vi "UHR-Fleezers Control (host) - Avogadro v3.vi"() -> ()   [LabVIEW 2014] (continued)
              }
            }
          }
          frame "Triggered" {
            n3649 = local read "Trap Trig. (FPGA)"() -> (w5268:bool)
            n3650 = Increment(x=w5271) -> (x+1=w5269:i32)
            n3651 = Greater Or Equal?(x=w5269, y="Fl. ON time (n)") -> (x >= y?=w5267:bool)
            n3652 = Select(t="Wait for trigger", s=w5267, f="Triggered" ("t")) -> (s? t:f=w5272:string)
            n3653 = And(x=w5267, y=w5268) -> (x .and. y?=w5264:bool)
            n3654 = case shown="True" w5264 {
              tunnel: w5266 -> [_ w5276]
              tunnel: w5265 -> [_ w5275]
              frame False {
              }
              frame True {
                n3655 = xnode "Read/Write Control"("FPGA VI Reference In"=w5276, "error in"=w5275, "FPGA Trap Trig"=TRUE) -> ()  [unwired: 2 out]
              }
            }
            n3656 = case shown="True" w5267 {
              frame False {
              }
              frame True {
                w5278 = FALSE ("Value (Signaling)")
                n3657 = local write "Triggered"(w5278) -> ()
                n3658 = local write "Waiting"(TRUE ("Waiting")) -> ()
                n3659 = property on="Vortran Laser ON" class="Bool (strict)"("Val(Sgnl)"=w5278) -> ()  [unwired: 2 in, 2 out]
              }
            }
          }
          frame "Do nothing" {
          }
          frame "Initialize", Default {
            n3660 = Increment(x=w5289) -> (x+1=w5293:i32)
            n3661 = Select(t=1, s=w5282, f=w5293) -> (s? t:f=w5283:i32)
            n3662 = feedback #23(w5291) -> (w5297:dbl[])
            n3663 = Build Array (concatenate)(w5291, w5297) -> (w5290:dbl[])
            n3664 = Greater Or Equal?(x=w5283, y="Wait to get offset (n)") -> (x >= y?=w5286:bool)
            n3665 = Select(t=w5291, s=w5282, f=w5290) -> (s? t:f=w5292:dbl[])
            n3666 = feedback-in #23(w5292) -> ()
            n3667 = call-poly <vilib>:"Mean.vi"("X"=w5292) -> ("mean"=w5287:dbl)  [unwired: 1 out]
            n3668 = local write "Mean T1 Position\nto compare (nm)"(w5287) -> ()
            n3669 = case shown="True" w5282 {
              tunnel: w5285 -> [_ w5303]
              tunnel: w5284 -> [_ w5302]
              frame False {
              }
              frame True {
                w5299 = FALSE ("FPGA Trap Trig")
                n3670 = xnode "Read/Write Control"("FPGA VI Reference In"=w5303, "error in"=w5302, "FPGA Trap Trig"=w5299) -> ("FPGA VI Reference Out"=w5301:T41, "error out"=w5300:errorcluster)
                n3671 = xnode "Read/Write Control"("FPGA VI Reference In"=w5301, "error in"=w5300, "TTrig?"=w5299) -> ()  [unwired: 2 out]
              }
            }
            n3672 = Select(t="Wait for trigger", s=w5286, f="Initialize") -> (s? t:f=w5294:string)
            n3673 = case shown="True" w5286 {
              tunnel: w5287 -> [_ w5306]
              tunnel: w5285 -> [_ w5315]
              tunnel: w5284 -> [_ w5314]
              frame False {
                n3674 = local write "Waiting"(FALSE ("Waiting")) -> ()
                "Initializing" <- TRUE ("Initializing")
              }
              frame True {
                n3675 = local read "Threshold (nm)"() -> (w5318:dbl)
                n3676 = local read "AOM X Cal (nm/MHz)"() -> (w5317:dbl)
                n3677 = Add(x=w5306, y=w5318) -> (x+y=w5319:dbl)
                n3678 = Divide(x=w5319, y=w5317) -> (x/y=w5316:dbl)
                n3679 = call "IR AOM freq to word.vi"("Frequency In (MHz)"=w5316) -> ("Frequency Word Out (double)"=w5313:dbl)
                n3680 = local write "Initializing"(FALSE ("Initializing")) -> ()
                n3681 = local write "Waiting"(TRUE ("Waiting")) -> ()
                n3682 = To Quad Integer(1:w5313) -> (0:w5312:i64)
                n3683 = xnode "Read/Write Control"("FPGA VI Reference In"=w5315, "error in"=w5314, "FPGA TTrig Thresh"=w5312) -> ("FPGA VI Reference Out"=w5309:T41, "error out"=w5308:errorcluster)
                n3684 = xnode "Read/Write Control"("FPGA VI Reference In"=w5309, "error in"=w5308, "FPGA Trap Trig"=TRUE) -> ()  [unwired: 2 out]
              }
            }
          }
        }
      }
    }
    n3685 = feedback-in #21(w4841) -> ()
    n3686 = feedback-in #22(w4838) -> ()
    n3687 = xnode ("Read/Write Control")("FPGA VI Reference In"=w4633, "error in"=w4900) -> ("FPGA VI Reference Out"=w4630:T41, "error out"=w4826:errorcluster, "AI2 Y Sum Set 1"=w4942:i16, "AI2 Y Sum Set 2"=w4941:i16, "AI1 X Set 1"=w4857:fxp<+/-,16,1>, "AI1 X Set 2"=w4856:fxp<+/-,16,1>, "Trap Pos FB Int Signal"=→"Trap Pos FB Int Signal":fxp<+/-,24,9>, "Trap Pos FB Int-Norm Signal"=→"Trap Pos FB Int-Norm Signal":fxp<+/-,16,1>, "Trap Pos FB Action"=w4850:i64, "Scanning"=→"AOD Scanning":bool, "Scan I"=→"AOD Scan I":u64, "Scanning MCL"=w4944:bool, "Scan I (MCL)"=→"MCL Scan I":u64, "Green FB Sum"=w4907:i16, "Trap Pos FB Action"=w4824:i64, "TTrig Fin Thresh"=w4820:i64, "Red FB Intensity"=w4812:i16, "Blue Intensity"=w4807:i16, "BD1 Frequency Out 1"=w4772:u64)
    "MCL Scanning" <- w4944
    "Trap Pos FB Action" <- w4850
    n3688 = Divide(x=w4812, y=3276.7) -> (x/y=w4811:dbl)
    "Red laser intensity (V)" <- w4811
    n3689 = Divide(x=w4807, y=3276.7) -> (x/y=w4806:dbl)
    "Blue laser intensity (V)" <- w4806
    n3690 = Divide(x=w4907, y=3276.7) -> (x/y=w4810:dbl)
    "Green laser intensity (V)" <- w4810
    n3691 = local read "FB Trig Integrate"() -> (w4818:u32)
    n3692 = Divide(x=w4824, y=w4818) -> (x/y=w4817:dbl)
    "TTrig Sig (Int)" <- w4817
    n3693 = Bundle(w4810, w4811, w4806) -> (→"Fluorescence laser intensities plot":cluster{dbl, dbl, dbl})  [unwired: 1 in]
    n3694 = Divide(x=w4820, y=w4818) -> (x/y=w4815:dbl)
    "TTrig Fin Thresh (Int)" <- w4815
    n3695 = local read "AOM X Cal (nm/MHz)"() -> (w4823:dbl)
    n3696 = local read "AI2 (V)"() -> (w4943:cluster{"Set 1":dbl, "Set 2":dbl})
    n3697 = Bundle By Name(cluster=w4943, "Set 1"=w4942, "Set 2"=w4941) -> (w4774:cluster{"Set 1":dbl, "Set 2":dbl})
    n3698 = Divide(x=w4850, y=327.67) -> (x/y=→"Action (%)":dbl)
    n3699 = case shown="True" "Semi Passive Mode" {
      tunnel: w4680 -> [_ w5091]
      frame False {
      }
      frame True {
        n3700 = local read "Target Force (pN)"() -> (w5089:dbl)
        n3701 = Less?(x="Jump Force (pN)", y=w5089) -> (x < y?=w5087:bool)
        n3702 = case shown="False" w5087 {
          tunnel: "Jump Force (pN)" -> [w5097 w5100]
          tunnel: w5091 -> [w5096 w5099]
          tunnel: [w5095 w5098] -> w5090
          frame False {
            n3703 = Less?(x=w5097, y=w5096) -> (x < y?=w5095:bool)
          }
          frame True {
            n3704 = Greater?(x=w5100, y=w5099) -> (0:w5098:bool)
          }
        }
        n3705 = case shown="False" w5090 {
          frame False {
            n3706 = local read "Trap Pos. FB ON"() -> (w5092:bool)
            n3707 = case shown="False" w5092 {
              frame False {
              }
              frame True {
                n3708 = property on="Trap Pos. FB ON" class="Bool (strict)"("Val(Sgnl)"=FALSE) -> ()  [unwired: 2 in, 2 out]
              }
            }
          }
          frame True {
            n3709 = property on="Trap Pos. FB ON" class="Bool (strict)"("Val(Sgnl)"=TRUE) -> ()  [unwired: 2 in, 2 out]
          }
        }
      }
    }
    n3710 = local read "Trap X (AI1)"() -> (w4870:T19)
    n3711 = call "IR AOM word double to freq.vi"("Frequency Word In (double)"=w4815) -> ("Frequency Out (MHz)"=w4814:dbl)
    n3712 = call "IR AOM word double to freq.vi"("Frequency Word In (double)"=w4817) -> ("Frequency Out (MHz)"=w4816:dbl)
    n3713 = Divide(x=w4774, y=3276.7) -> (x/y=w4939:cluster{"Set 1":dbl, "Set 2":dbl})
    n3714 = Multiply(x=w4816, y=w4823) -> (x*y=w4822:dbl)
    "TTrig Sig (nm)" <- w4822
    n3715 = Multiply(x=w4814, y=w4823) -> (x*y=w4821:dbl)
    "TTrig Fin Thresh (nm)" <- w4821
    n3716 = local write "AI2 (V)"(w4939) -> ()
    n3717 = Bundle(cluster=w4870, "Trap 1"=w4857, "Trap 2"=w4856) -> (→"Trap X (AI1)":T19)
    n3718 = local read "Trap Pos. FB ON"() -> (w4765:bool)
    n3719 = local read "Dynamic Force FB (ronen)"() -> (w4766:bool)
    n3720 = Bundle(w4822, w4821) -> (→"TTrig":cluster{dbl, dbl})  [unwired: 1 in]
    n3721 = Compound Arithmetic op=AND(w4766, "Real time Offset file correction for setpoint", w4765) -> (w4767:bool)
    n3722 = case shown="True" w4767 {
      tunnel: w4772 -> [_ _]
      tunnel: w4703 -> [_ w5119]
      tunnel: w4630 -> [_ w5102]
      frame False {
      }
      frame True {
        # "Changed by Ronen - real time update of set point\naccording to offset file"
        n3723 = local read "T1 calibration"() -> (w5114:T12)
        n3724 = local read "Offset file step size"() -> (w5121:dbl)
        n3725 = local read "Setpoint offset\ncorrection values"() -> (w5118:dbl[])
        n3726 = Multiply(x="Target Force (pN)", y=2.0) -> (x*y=w5115:dbl)
        n3727 = local read "Negate Diff?"() -> (w5103:bool)
        n3728 = Unbundle By Name(w5114) -> ("alpha_x (nm/V)"=w5113:dbl, "kappa_x (pN/nm)"=w5112:dbl)
        n3729 = Divide(x=w5119, y=w5121) -> (x/y=w5122:dbl)
        n3730 = To Long Integer(number=w5122) -> (32bit integer=w5120:i32)
        n3731 = Index Array(array=w5118, index=w5120) -> (element=w5105:dbl)
        n3732 = Multiply(x=w5113, y=w5112) -> (x*y=w5111:dbl)
        n3733 = Select(t=1, s=w5103, f=-1) -> (s? t:f=w5106:i32)
        n3734 = Divide(x=w5115, y=w5111) -> (x/y=w5110:dbl)
        n3735 = Multiply(x=w5106, y=w5105) -> (x*y=w5104:dbl)
        n3736 = Add(x=w5110, y=w5104) -> (x+y=w5109:dbl)
        n3737 = To Fixed-Point(number=w5109) -> (fixed-point=w5101:fxp<+/-,16,1>)  [unwired: 1 in]
        "Actual Setpoint" <- w5101
        n3738 = xnode "Read/Write Control"("FPGA VI Reference In"=w5102, "Trap Pos. FB SP"=w5101) -> ()  [unwired: 1 in, 2 out]
      }
    }
    n3739 = local read "All FB On/Off"() -> (w4773:bool)
    n3740 = case shown="True" w4773 {
      tunnel: w4630 -> [_ w5146]
      frame False {
      }
      frame True {
        n3741 = local read "X RF Amplitude Limits (%)"() -> (w5145:T27)
        n3742 = xnode "Read/Write Control"("FPGA VI Reference In"=w5146) -> ("BD1 amplitude 1 out"=w5137:u16, "BD1 amplitude 2 out"=w5129:u16)  [unwired: 1 in, 2 out]
        n3743 = Unbundle By Name(w5145) -> ("Maximum"=w5128:dbl)
        n3744 = Scale By Power Of 2(n=i16 12, x=ext 1.0) -> (x*2^n=w5141:ext)
        n3745 = Scale By Power Of 2(n=i16 12, x=ext 1.0) -> (x*2^n=w5133:ext)
        n3746 = Subtract(x=w5141, y=ext 1.0) -> (x-y=w5143:ext)
        n3747 = Subtract(x=w5133, y=ext 1.0) -> (x-y=w5131:ext)
        n3748 = Multiply(x=w5137, y=ext 100.0) -> (x*y=w5144:ext)
        n3749 = Multiply(x=w5129, y=ext 100.0) -> (x*y=w5130:ext)
        n3750 = Divide(x=w5144, y=w5143) -> (x/y=w5124:ext)
        "T1 feedback amplitude" <- w5124
        n3751 = Divide(x=w5130, y=w5131) -> (x/y=w5123:ext)
        "T2 feedback amplitude" <- w5123
        n3752 = Greater?(x=w5123, y=w5128) -> (0:w5126:bool)
        n3753 = Greater?(x=w5124, y=w5128) -> (0:w5127:bool)
        n3754 = Or(x=w5127, y=w5126) -> (x .or. y?=w5125:bool)
        n3755 = case shown="True" w5125 {
          frame False {
          }
          frame True {
            n3756 = property on="All FB On/Off" class="Bool (strict)"("Val(Sgnl)"=FALSE) -> ()  [unwired: 2 in, 2 out]
          }
        }
      }
    }
    n3757 = flat-sequence "To save data" {
      tunnel: [w5865] -> w4962
      tunnel: [w5866] -> w4961
      tunnel: w4924 -> [w5859]
      tunnel: w4646 -> [w5863]
      tunnel: ["Save Calibration"] -> w4936
      tunnel: w4755 -> [w5862]
      tunnel: [w5855] -> w4933
      tunnel: [w5852] -> w4932
      tunnel: [w5849] -> w4931
      tunnel: w4923 -> [w5851]
      tunnel: w4711 -> [w5845]
      tunnel: [w5845] -> w4894
      tunnel: ["Start Saving"] -> w4879
      tunnel: [w5840] -> w4846
      tunnel: [w5839] -> w4845
      tunnel: [w5836] -> w4778
      tunnel: [w5832] -> w4771
      tunnel: w4962 -> [w6199]
      tunnel: w4961 -> [w6198]
      tunnel: w4756 -> [w6197]
      tunnel: w4936 -> [w6196]
      tunnel: w4933 -> [w6194]
      tunnel: w4932 -> [w6193]
      tunnel: w4931 -> [w6192]
      tunnel: w4750 -> [w6191]
      tunnel: w4754 -> [w6190]
      tunnel: w4894 -> [w6189]
      tunnel: w4879 -> [w6188]
      tunnel: w4634 -> [w6187]
      tunnel: w4805 -> [w6186]
      tunnel: w4846 -> [w6185]
      tunnel: w4845 -> [w6184]
      tunnel: w4707 -> [w6183]
      tunnel: w4716 -> [w6182]
      tunnel: w4753 -> [w6181]
      tunnel: w4778 -> [w6180]
      tunnel: w4771 -> [w6179]
      frame #0 {
        # "Changed by Ronen - we don't have a database so we disabled this"
        n3758 = Or(x="Save N Sets", y="Start Saving") -> (x .or. y?=w5846:bool)
        n3759 = To Double Precision Float(number=w5862) -> (double precision float=w5856:dbl)
        n3760 = Build Array(w5846, "Save Calibration", w5859, w5851, "Flow Cal") -> (w5861:bool[])
        n3761 = Compound Arithmetic op=OR("Save Calibration", w5859, w5846, w5851, "Flow Cal") -> (w5864:bool)
        n3762 = Boolean Array To Number(Boolean array=w5861) -> (number=w5858:u32)
        n3763 = feedback #24(FALSE ("Save APD Data\nwith Trap Data")) -> (w5841:bool)
        n3764 = feedback #25(refnum<k0> refnum) -> (w5867:refnum<file>)
        n3765 = feedback #26(FALSE ("Save APD Data\nwith Trap Data")) -> (w5850:bool)
        n3766 = feedback #27(0) -> (w5869:i32)
        n3767 = feedback #28() -> (w5857:u32)  [unwired: 1 out]
        n3768 = feedback #29(refnum<k0> refnum) -> (w5837:refnum<file>)
        n3769 = feedback #30(refnum<k0> refnum) -> (w5843:refnum<file>)
        n3770 = feedback #31(refnum<k0> refnum) -> (w5833:refnum<file>)
        n3771 = feedback #32(refnum<k0> refnum) -> (w5853:refnum<file>)
        n3772 = case shown="True" w5864 {
          tunnel: [w5878 1] -> w5865
          tunnel: w5869 -> [w5880 _]
          tunnel: [w5879 w5912] -> w5866
          tunnel: w5867 -> [w5879 _]
          tunnel: w5863 -> [_ w5930]
          tunnel: w5856 -> [_ w5928]
          tunnel: w5858 -> [_ w5931]
          tunnel: [w5877 w5911] -> w5855
          tunnel: w5857 -> [w5877 _]
          tunnel: [w5876 w5909] -> w5852
          tunnel: w5853 -> [w5876 _]
          tunnel: [w5875 w5908] -> w5849
          tunnel: w5850 -> [w5875 _]
          tunnel: "Start Saving" -> [_ w5906]
          tunnel: w5845 -> [_ w5905]
          tunnel: [w5874 w5898] -> w5839
          tunnel: w5843 -> [w5874 _]
          tunnel: [w5873 w5897] -> w5840
          tunnel: w5841 -> [w5873 _]
          tunnel: [w5872 w5883] -> w5836
          tunnel: w5837 -> [w5872 _]
          tunnel: [w5871 w5881] -> w5832
          tunnel: w5833 -> [w5871 _]
          frame False {
            n3773 = Increment(x=w5880) -> (x+1=w5878:i32)
          }
          frame True {
            w5882 = FALSE ("Start Saving")
            w5907 = 10.0  # File Version
            w5914 = FALSE ("prepend array or string size? (T)")
            w5913 = T54."big-endian, network order" ("byte order (0:big-endian, network order)")
            # "RG added position values of traps in the saved\nfile for AOD rasters and time series."
            # "Ronen Changed the create file - changed data folder to c:\\Data"
            # "Save trap position\ndata"
            n3774 = Array Size(array=w5905) -> (size(s)=w5904:i32)
            n3775 = To Double Precision Float(number=w5904) -> (double precision float=w5903:dbl)
            n3776 = local read "BD 1 Frequency 1 (MHz)"() -> (w5927:dbl)
            n3777 = local read "BD 2 Frequency 1 (MHz)"() -> (w5926:dbl)
            n3778 = local read "BD 1 Frequency 2 (MHz)"() -> (w5925:dbl)
            n3779 = local read "BD 2 Frequency 2 (MHz)"() -> (w5924:dbl)
            n3780 = local read "BD 1 Frequency 3 (MHz)"() -> (w5923:dbl)
            n3781 = local read "BD 2 Frequency 3 (MHz)"() -> (w5922:dbl)
            n3782 = local write "Flow Cal"(w5882) -> ()
            n3783 = local write "Save Calibration"(w5882) -> ()
            n3784 = local write "Start Saving"(w5882) -> ()
            n3785 = Build Array("Save APD Data\nwith Trap Data", "Save Trap Pos. Data") -> (w5900:bool[])
            n3786 = Boolean Array To Number(Boolean array=w5900) -> (number=w5899:u32)
            n3787 = Build Array(w5927, w5926, w5925, w5924, w5923, w5922) -> (w5921:dbl[])
            n3788 = case shown="1, Default" w5931 {
              tunnel: w5930 -> [w6037 w6064 w6096 w6134 w6171]
              tunnel: w5903 -> [w6042 w6071 w6116 w6153 w6176]
              tunnel: w5928 -> [w6041 w6070 w6115 w6152 w6175]
              tunnel: [w6038 w6066 w6107 w6144 w6172] -> w5919
              tunnel: [w6029 "Cal sets to save" w6097 w6135 w6158] -> w5911
              tunnel: w5921 -> [w6039 w6067 w6109 w6146 w6173]
              tunnel: "Save APD Data\nwith Trap Data" -> [w6036 w6053 w6094 w6132 w6170]
              tunnel: [w6036 w6051 w6094 w6132 w6170] -> w5908
              tunnel: w5907 -> [w6032 w6060 w6092 w6130 w6166]
              tunnel: w5906 -> [w6031 _ _ _ _]
              tunnel: [w6022 w6059 w6091 w6120 w6165] -> w5897
              tunnel: "Save Trap Pos. Data" -> [w6022 w6058 w6091 w6120 w6165]
              tunnel: w5899 -> [w6021 w6057 w6090 w6119 w6164]
              frame 1, Default {
                # "timeseries"
                n3789 = case shown="True" "Profile" {
                  tunnel: [w6045 w6049] -> w6026
                  tunnel: [w6045 w6048] -> w6025
                  tunnel: [w6045 w6047] -> w6024
                  tunnel: [w6045 w6046] -> w6023
                  frame False {
                    w6045 = 0.0 ("f")
                  }
                  frame True {
                    n3790 = local read "Current Position"() -> (w6050:cluster{dbl, dbl, dbl})
                    n3791 = local read "Y change (mm)"() -> (w6046:dbl)
                    n3792 = Unbundle(w6050) -> (w6049:dbl, w6048:dbl, w6047:dbl)
                  }
                }
                n3793 = local read "Save ave N"() -> (w6044:dbl)
                n3794 = local read "AOM X Cal (nm/MHz)"() -> (w6020:dbl)
                n3795 = local read "Piezo Trap X cal (nm/V)"() -> (w6019:dbl)
                n3796 = local read "Piezo Trap Y cal (nm/V)"() -> (w6018:dbl)
                n3797 = local read "Piezo trap x\noffset (V)"() -> (w6017:dbl)
                n3798 = local read "Piezo trap y\noffset (V)"() -> (w6016:dbl)
                n3799 = To Double Precision Float(number=w6021) -> (double precision float=w6035:dbl)
                n3800 = Multiply(x=w6044, y=w6037) -> (x*y=w6043:dbl)
                n3801 = Build Array(w6032, w6037, w6043, w6042, w6041, 0.0 ("f")) -> (w6040:dbl[])
                n3802 = Build Array(w6035, w6026, w6025, w6024, w6023) -> (w6033:dbl[])
                n3803 = Build Array(w6020, w6019, w6018, w6017, w6016) -> (w6015:dbl[])
                n3804 = Select(t=u32 4000000000, s=w6031, f="N sets to save") -> (s? t:f=w6029:u32)
                n3805 = Build Array (concatenate)(w6040, w6039, w6033, w6015) -> (w6038:dbl[])
              }
              frame 2 {
                w6062 = 0.0 ("f")
                w6052 = FALSE ("Save APD Data\nwith Trap Data")
                # "For diagnostics save trap position\ndata during cal"
                # "calibration"
                n3806 = Boolean To (0,1)(Boolean=w6052) -> (0, 1=w6056:i16)
                n3807 = Select(t=w6053, s="Save trap pos with cal", f=w6052) -> (s? t:f=w6051:bool)
                n3808 = Select(t=w6058, s="Save trap pos with cal", f=w6052) -> (s? t:f=w6059:bool)
                n3809 = Select(t=w6057, s="Save trap pos with cal", f=w6056) -> (s? t:f=w6055:u32)
                n3810 = To Double Precision Float(number=w6055) -> (double precision float=w6063:dbl)
                n3811 = Build Array(w6060, w6064, w6064, w6071, w6070, 1.0 ("t")) -> (w6068:dbl[])
                n3812 = Build Array(w6063, w6062, w6062, w6062, w6062) -> (w6061:dbl[])
                n3813 = Build Array (concatenate)(w6068, w6067, w6061) -> (w6066:dbl[])
                "Calibrating Trap..." <- TRUE ("Calibrating...")
              }
              frame 4 {
                # "scan dir (x/y = 0/1)"
                # "cycles/step"
                # "n scans (f/b)"
                # "steps"
                # "freq. range"
                # "AOD raster scan"
                n3814 = local read "MCL offset scanning range (V)"() -> (w6087:T4)
                n3815 = local read "Multiple-MCL offset?"() -> (w6082:bool)
                n3816 = local read "Piezo Trap Y cal (nm/V)"() -> (w6073:dbl)
                n3817 = local read "AOM X Cal (nm/MHz)"() -> (w6075:dbl)
                n3818 = local read "Piezo Trap X cal (nm/V)"() -> (w6076:dbl)
                n3819 = local read "Piezo trap x\noffset (V)"() -> (w6077:dbl)
                n3820 = local read "Piezo trap y\noffset (V)"() -> (w6078:dbl)
                n3821 = local read "Number of F/B Scans (AOD)"() -> (w6101:u16)
                n3822 = Boolean To (0,1)(Boolean="Offset raster?") -> (0, 1=w6080:i16)
                n3823 = call "Make Trap3 position array.vi"("MCL offset scanning range (V)"=w6087) -> ("X Data points"=w6086:u64, "Y data points"=w6085:u64)  [unwired: 3 out]
                n3824 = Boolean To (0,1)(Boolean=w6082) -> (0, 1=w6089:i16)
                n3825 = local read "Cycles/step (AOD)"() -> (w6103:u64)
                n3826 = local read "Scan Range (MHz)"() -> (w6106:dbl)
                n3827 = local read "Scan steps (AOD)"() -> (w6105:u64)
                n3828 = local read "Scan BD"() -> (w6113:bool)
                n3829 = To Double Precision Float(number=w6089) -> (double precision float=w6088:dbl)
                n3830 = local read "Save ave N"() -> (w6118:dbl)
                n3831 = To Double Precision Float(number=w6085) -> (double precision float=w6083:dbl)
                n3832 = Build Array(w6075, w6076, w6073, w6077, w6078) -> (w6074:dbl[])
                n3833 = To Double Precision Float(number=w6086) -> (double precision float=w6084:dbl)
                n3834 = Boolean To (0,1)(Boolean=w6113) -> (0, 1=w6112:i16)
                n3835 = To Double Precision Float(number=w6080) -> (double precision float=w6079:dbl)
                n3836 = To Double Precision Float(number=w6101) -> (double precision float=w6100:dbl)
                n3837 = To Double Precision Float(number=w6105) -> (double precision float=w6104:dbl)
                n3838 = To Double Precision Float(number=w6103) -> (double precision float=w6102:dbl)
                n3839 = To Double Precision Float(number=w6112) -> (double precision float=w6111:dbl)
                n3840 = Multiply(x=w6118, y=w6096) -> (x*y=w6117:dbl)
                n3841 = To Double Precision Float(number=w6090) -> (double precision float=w6095:dbl)
                n3842 = local read "N sets should be saved"() -> (w6098:dbl)
                n3843 = Build Array(w6095, w6088, w6084, w6083, w6079) -> (w6093:dbl[])
                n3844 = Build Array(w6111, w6106, w6104, w6102, w6100) -> (w6108:dbl[])
                n3845 = Build Array(w6092, w6096, w6117, w6116, w6115, 2.0 ("t")) -> (w6110:dbl[])
                n3846 = Build Array (concatenate)(w6110, w6109, w6093, w6108, w6074) -> (w6107:dbl[])
                n3847 = Round Toward +Infinity(x=w6098) -> (ceil(x): smallest int >= x=w6099:dbl)
                n3848 = To Unsigned Long Integer(number=w6099) -> (unsigned 32bit integer=w6097:u32)
              }
              frame 8 {
                w6127 = 0.0 ("f")
                # "MCL raster scan"
                n3849 = local read "Number of scans (MCL)"() -> (w6122:u64)
                n3850 = local read "2D or 1D Scan"() -> (w6124:bool)
                n3851 = local read "Scan lines (y)"() -> (w6121:u64)
                n3852 = local read "Scan Range (V)\n(of steps)"() -> (w6143:dbl)
                n3853 = local read "Fast Scan Dir"() -> (w6150:bool)
                n3854 = local read "Cycles/step (MCL)"() -> (w6140:u64)
                n3855 = local read "Scan steps (MCL)"() -> (w6142:u64)
                n3856 = Select(t=w6121, s=w6124, f=w6122) -> (s? t:f=w6123:u64)
                n3857 = Boolean To (0,1)(Boolean=w6124) -> (0, 1=w6126:i16)
                n3858 = local read "Save ave N"() -> (w6155:dbl)
                n3859 = local read "Initial X"() -> (w6129:dbl)
                n3860 = local read "Initial Y"() -> (w6128:dbl)
                n3861 = To Double Precision Float(number=w6126) -> (double precision float=w6125:dbl)
                n3862 = Boolean To (0,1)(Boolean=w6150) -> (0, 1=w6149:i16)
                n3863 = To Double Precision Float(number=w6123) -> (double precision float=w6138:dbl)
                n3864 = To Double Precision Float(number=w6142) -> (double precision float=w6141:dbl)
                n3865 = To Double Precision Float(number=w6140) -> (double precision float=w6139:dbl)
                n3866 = To Double Precision Float(number=w6149) -> (double precision float=w6148:dbl)
                n3867 = Multiply(x=w6155, y=w6134) -> (x*y=w6154:dbl)
                n3868 = To Double Precision Float(number=w6119) -> (double precision float=w6133:dbl)
                n3869 = local read "N sets should be saved (MCL)"() -> (w6136:dbl)
                n3870 = Build Array(w6133, w6125, w6127, w6127, w6127) -> (w6131:dbl[])
                n3871 = Build Array(w6148, w6143, w6141, w6139, w6138, w6129, w6128) -> (w6145:dbl[])
                n3872 = Build Array(w6130, w6134, w6154, w6153, w6152, 3.0 ("t")) -> (w6147:dbl[])
                n3873 = Round Toward +Infinity(x=w6136) -> (ceil(x): smallest int >= x=w6137:dbl)
                n3874 = Build Array (concatenate)(w6147, w6146, w6131, w6145) -> (w6144:dbl[])
                n3875 = To Unsigned Long Integer(number=w6137) -> (unsigned 32bit integer=w6135:u32)
              }
              frame 16 {
                w6157 = 0.0
                # "Flow calibration - added by Ronen: Number\nof saved sets is distance (1 mm) divided by \nspeed +1.5 spare second divided by the time of\nset measurement, 0.2 sec for 2 set interlace"
                # "timeseries"
                n3876 = local read "Save ave N"() -> (w6178:dbl)
                n3877 = Reciprocal(x=0.0) -> (1/x=w6163:dbl)
                n3878 = Add(x=w6163, y=1.5) -> (x+y=w6161:dbl)
                n3879 = Multiply(x=w6178, y=w6171) -> (x*y=w6177:dbl)
                n3880 = Divide(x=w6161, y=0.2) -> (x/y=w6159:dbl)
                n3881 = To Double Precision Float(number=w6164) -> (double precision float=w6169:dbl)
                n3882 = To Unsigned Long Integer(number=w6159) -> (unsigned 32bit integer=w6158:u32)
                n3883 = Build Array(w6166, w6171, w6177, w6176, w6175, 4.0 ("f")) -> (w6174:dbl[])
                n3884 = Build Array(w6169, w6157, w6157, w6157, w6157) -> (w6167:dbl[])
                n3885 = Build Array (concatenate)(w6174, w6173, w6167) -> (w6172:dbl[])
              }
            }
            n3886 = local read "Index"() -> (w5936:dbl)
            n3887 = call "Create new save file.vi"("Insert"="", "Ext"=".dat", "Index In"=w5936) -> ("Path Out"=w5885:path, "Index Out"=w5910:dbl)
            n3888 = local write "Save file name"(w5885) -> ()
            n3889 = local write "Index"(w5910) -> ()
            n3890 = local write "Save index"(w5910) -> ()
            n3891 = case shown="True" "Save Event Log?" {
              tunnel: w5885 -> [_ w5950]
              tunnel: [refnum<k0> refnum w5949] -> w5883
              frame False {
              }
              frame True {
                (unwired) FALSE ("prepend array or string size? (T)")
                n3892 = Path To String(path=w5950) -> (string=w5961:string)
                n3893 = String Length(string=w5961) -> (length=w5960:i32)
                n3894 = Subtract(x=w5960, y=4) -> (x-y=w5958:i32)
                n3895 = String Subset(string=w5961, length (rest)=w5958) -> (substring=w5957:string)  [unwired: 1 out]
                n3896 = Concatenate Strings(w5957, "_log.txt" ("string")) -> (w5955:string)
                n3897 = String To Path(string=w5955) -> (path=w5951:path)
                n3898 = Open/Create/Replace File(file path (use dialog)=w5951, operation (0:open)=T53."create", access (0:read/write)=enum16{"read/write", "read-only", "write-only"}."write-only") -> (refnum out=w5952:refnum<file>)  [unwired: 1 in, 4 out]
                n3899 = Deny Access(7:w5952) -> (3:w5949:refnum<file>)  [unwired: 1 in, 2 out]
                n3900 = call "write to event log.vi"("log file ref"=w5949, "time"=0.0, "input string"="start log") -> ()  [unwired: 8 in]
              }
            }
            "log file ref" <- w5883
            n3901 = Array Size(array=w5919) -> (size(s)=w5920:i32)
            n3902 = Open/Create/Replace File(file path (use dialog)=w5885, operation (0:open)=T53."create", access (0:read/write)=enum16{"read/write", "read-only", "write-only"}."write-only") -> (refnum out=w5933:refnum<file>)  [unwired: 1 in, 4 out]
            n3903 = local write "Saving..."(TRUE ("Saving...")) -> ()
            n3904 = To Double Precision Float(number=w5920) -> (double precision float=w5918:dbl)
            n3905 = String Length(string="Comment (data description)") -> (length=w5917:i32)
            n3906 = To Double Precision Float(number=w5917) -> (double precision float=w5916:dbl)
            n3907 = Deny Access(7:w5933) -> (3:w5932:refnum<file>)  [unwired: 1 in, 2 out]
            n3908 = Build Array (concatenate)(w5918, w5919, w5916) -> (w5895:dbl[])
            n3909 = case "If fluorescence data to be saved" shown="True" w5908 {
              tunnel: w5885 -> [_ w6014]
              tunnel: [w5984 w5997] -> w5909
              tunnel: [w5984 w5985] -> w5881
              frame False {
                w5984 = refnum<k0> refnum
              }
              frame True {
                w5996 = 0.0
                w5989 = T53."create" ("operation (0:open)")
                w5990 = enum16{"read/write", "read-only", "write-only"}."write-only" ("access (0:read/write)")
                n3910 = local read "APD Integration Time (s)"() -> (w6002:dbl)
                n3911 = local read "N APD Samp/step"() -> (w5995:dbl)
                n3912 = local read "Number of APDs"() -> (w5994:u8)
                n3913 = Path To String(path=w6014) -> (string=w6013:string)
                n3914 = String Length(string=w6013) -> (length=w6012:i32)
                n3915 = Subtract(x=w6012, y=4) -> (x-y=w6010:i32)
                n3916 = String Subset(string=w6013, length (rest)=w6010) -> (substring=w5993:string)  [unwired: 1 out]
                n3917 = Build Array(w6002, w5995, w5994, w5996, w5996, w5996, w5996, w5996) -> (w5999:dbl[])
                n3918 = Concatenate Strings(w5993, "_green.dat") -> (w5991:string)
                n3919 = Concatenate Strings(w5993, "_fl.dat" ("string")) -> (w6008:string)
                n3920 = Array Size(array=w5999) -> (size(s)=w6001:i32)
                n3921 = String To Path(string=w6008) -> (path=w6006:path)
                n3922 = Open/Create/Replace File(file path (use dialog)=w6006, operation (0:open)=w5989, access (0:read/write)=w5990) -> (refnum out=w6007:refnum<file>)  [unwired: 1 in, 4 out]
                n3923 = Deny Access(7:w6007) -> (3:w6003:refnum<file>)  [unwired: 1 in, 2 out]
                n3924 = String To Path(string=w5991) -> (path=w5988:path)
                n3925 = To Double Precision Float(number=w6001) -> (double precision float=w6000:dbl)
                n3926 = Build Array (concatenate)(w6000, w5999) -> (w5998:dbl[])
                n3927 = Write to Binary File(file (use dialog)=w6003, data=w5998, 5:FALSE ("prepend array or string size? (T)"), 9:T54."big-endian, network order" ("byte order (0:big-endian, network order)")) -> (refnum out=w5997:refnum<file>)  [unwired: 1 in, 3 out]
                n3928 = Open/Create/Replace File(file path (use dialog)=w5988, operation (0:open)=w5989, access (0:read/write)=w5990) -> (refnum out=w5986:refnum<file>, error out=w5987:errorcluster)  [unwired: 3 in, 1 out]
                n3929 = Deny Access(4:w5987, 7:w5986) -> (3:w5985:refnum<file>)  [unwired: 1 in, 1 out]
              }
            }
            n3930 = case shown="True" w5897 {
              tunnel: w5885 -> [_ w5969]
              tunnel: [refnum<k0> refnum w5968] -> w5898
              frame False {
              }
              frame True {
                w5964 = 0.0 ("element")
                n3931 = Path To String(path=w5969) -> (string=w5983:string)
                n3932 = Build Array(w5964, w5964, w5964, w5964, w5964, w5964, w5964, w5964) -> (w5965:dbl[])
                n3933 = String Length(string=w5983) -> (length=w5982:i32)
                n3934 = Subtract(x=w5982, y=4) -> (x-y=w5980:i32)
                n3935 = Array Size(array=w5965) -> (size(s)=w5967:i32)
                n3936 = String Subset(string=w5983, length (rest)=w5980) -> (substring=w5979:string)  [unwired: 1 out]
                n3937 = To Double Precision Float(number=w5967) -> (double precision float=w5966:dbl)
                n3938 = Concatenate Strings(w5979, "_pos.dat" ("string")) -> (w5977:string)
                n3939 = Build Array (concatenate)(w5966, w5965) -> (w5963:dbl[])
                n3940 = String To Path(string=w5977) -> (path=w5973:path)
                n3941 = Open/Create/Replace File(file path (use dialog)=w5973, operation (0:open)=T53."create", access (0:read/write)=enum16{"read/write", "read-only", "write-only"}."write-only") -> (refnum out=w5974:refnum<file>)  [unwired: 1 in, 4 out]
                n3942 = Deny Access(7:w5974) -> (3:w5970:refnum<file>)  [unwired: 1 in, 2 out]
                n3943 = Write to Binary File(file (use dialog)=w5970, data=w5963, 5:FALSE ("prepend array or string size? (T)"), 9:T54."big-endian, network order" ("byte order (0:big-endian, network order)")) -> (refnum out=w5968:refnum<file>)  [unwired: 1 in, 3 out]
              }
            }
            n3944 = Write to Binary File(file (use dialog)=w5932, data=w5895, 5:w5914, 9:w5913) -> (refnum out=w5915:refnum<file>)  [unwired: 1 in, 3 out]
            n3945 = Write to Binary File(file (use dialog)=w5915, data="Comment (data description)", 5:w5914, 9:w5913) -> (refnum out=w5912:refnum<file>)  [unwired: 1 in, 3 out]
            n3946 = local read "connection reference"() -> (w5896:T28)
            n3947 = Bundle("Comment (data description)"="Comment (data description)", "Channel 1 Buffer"="Channel 1 Buffer", "Channel 2 Buffer"="Channel 2 Buffer", "Channel 3 Buffer"="Channel 3 Buffer", "Title"="Title", "DNA Construct"="DNA Construct", "Bead diameter"="Bead diameter", "Name"="Name") -> (w5886:T75)  [unwired: 1 in]
            n3948 = disable-structure shown="Disabled" {
              disable-tunnel: w5896 -> [w5944 _]
              disable-tunnel: w5895 -> [w5942 _]
              disable-tunnel: w5886 -> [w5941 _]
              disable-tunnel: w5885 -> [w5940 _]
              frame Disabled {
                n3949 = call "MattFileCreator-v9.vi"("Comments"=w5941, "Input Array"=w5942, "File path"=w5940, "table"="labview", "connection reference"=w5944) -> ("connection reference out"=w5943:T28)  [unwired: 5 in, 1 out]
                n3950 = local write "connection reference"(w5943) -> ()
              }
              frame Enabled {
              }
            }
          }
        }
        n3951 = feedback-in #24(w5840) -> ()
        n3952 = feedback-in #25(w5866) -> ()
        n3953 = feedback-in #26(w5849) -> ()
        n3954 = feedback-in #27(w5865) -> ()
        n3955 = feedback-in #28(w5855) -> ()
        n3956 = feedback-in #29(w5836) -> ()
        n3957 = feedback-in #30(w5839) -> ()
        n3958 = feedback-in #31(w5832) -> ()
        n3959 = feedback-in #32(w5852) -> ()
      }
      frame #1 {
        n3960 = local read "Saving..."() -> (w6195:bool)
        n3961 = case shown="True" w6195 {
          tunnel: w6199 -> [_ w6213]
          tunnel: w6198 -> [_ w6227]
          tunnel: w6197 -> [_ w6223]
          tunnel: w6196 -> [_ w6222]
          tunnel: w6194 -> [_ w6221]
          tunnel: w6193 -> [_ w6216]
          tunnel: w6192 -> [_ w6215]
          tunnel: w6191 -> [_ w6214]
          tunnel: w6190 -> [_ w6212]
          tunnel: w6189 -> [_ w6210]
          tunnel: w6188 -> [_ w6209]
          tunnel: w6187 -> [_ w6208]
          tunnel: w6186 -> [_ w6207]
          tunnel: w6185 -> [_ w6206]
          tunnel: w6184 -> [_ w6205]
          tunnel: w6183 -> [_ w6204]
          tunnel: w6182 -> [_ w6203]
          tunnel: w6181 -> [_ w6202]
          tunnel: w6180 -> [_ w6201]
          tunnel: w6179 -> [_ w6200]
          frame False {
          }
          frame True {
            n3962 = Multiply(x=w6213, y=w6212) -> (x*y=→"Time (s)":dbl)
            n3963 = Less Or Equal?(x=w6213, y=w6221) -> (x <= y?=w6225:bool)
            n3964 = Compound Arithmetic op=OR("Stop Saving", "Abort save 2") -> (w6217:bool)
            n3965 = Not(x=w6217) -> (.not. x?=w6226:bool)
            n3966 = And(x=w6225, y=w6226) -> (x .and. y?=w6224:bool)
            n3967 = case shown="True" w6224 {
              tunnel: w6227 -> [w6237 w6338]
              tunnel: [0.0 w6341] -> w6220
              tunnel: w6213 -> [_ w6339]
              tunnel: w6221 -> [_ w6340]
              tunnel: w6223 -> [_ w6335]
              tunnel: w6222 -> [_ _]
              tunnel: w6216 -> [w6235 w6328]
              tunnel: w6215 -> [w6234 w6329]
              tunnel: w6214 -> [_ w6327]
              tunnel: w6210 -> [_ w6326]
              tunnel: w6209 -> [_ w6244]
              tunnel: w6208 -> [_ w6319]
              tunnel: w6207 -> [_ w6266]
              tunnel: w6206 -> [w6231 w6283]
              tunnel: w6205 -> [w6232 w6282]
              tunnel: w6204 -> [_ w6279]
              tunnel: w6203 -> [_ w6277]
              tunnel: w6202 -> [_ w6243]
              tunnel: w6201 -> [w6230 _]
              tunnel: w6200 -> [w6228 w6242]
              frame False {
                w6233 = FALSE
                n3968 = Close File(refnum=w6237) -> ()  [unwired: 1 in, 2 out]
                n3969 = case shown="True" w6234 {
                  tunnel: w6235 -> [_ w6241]
                  tunnel: w6228 -> [_ w6240]
                  frame False {
                  }
                  frame True {
                    n3970 = Close File(refnum=w6241) -> ()  [unwired: 1 in, 2 out]
                    n3971 = Close File(refnum=w6240) -> ()  [unwired: 1 in, 2 out]
                  }
                }
                n3972 = case shown="True" w6231 {
                  tunnel: w6232 -> [_ w6239]
                  frame False {
                  }
                  frame True {
                    n3973 = Close File(refnum=w6239) -> ()  [unwired: 1 in, 2 out]
                  }
                }
                n3974 = local read "Save Event Log?"() -> (w6229:bool)
                n3975 = case shown="True" w6229 {
                  tunnel: w6230 -> [_ w6238]
                  frame False {
                  }
                  frame True {
                    n3976 = Close File(refnum=w6238) -> ()  [unwired: 1 in, 2 out]
                  }
                }
                n3977 = local write "Raster Scanning..."(w6233) -> ()
                n3978 = local write "Calibrating Trap..."(w6233) -> ()
                n3979 = call <vilib>:"Beep.vi"() -> ()  [unwired: 3 in, 9 out]
                n3980 = local write "Stop Saving"(w6233) -> ()
                "Saving..." <- w6233
              }
              frame True {
                n3981 = local read "Calibrating Trap..."() -> (w6330:bool)
                n3982 = case "Write fl. data" shown="True" w6329 {
                  tunnel: w6328 -> [_ w6371]
                  tunnel: w6327 -> [_ w6370]
                  tunnel: w6242 -> [_ w6364]
                  frame False {
                  }
                  frame True {
                    w6363 = FALSE ("prepend array or string size? (T)")
                    w6365 = T54."big-endian, network order" ("byte order (0:big-endian, network order)")
                    n3983 = property on="Vortran Laser ON" class="Bool (strict)"() -> ("Value"=w6369:bool)  [unwired: 2 in, 2 out]
                    n3984 = property on="Green Intensity % (FB OFF)" class="DigNum (strict)"() -> ("Value"=w6368:dbl)  [unwired: 2 in, 2 out]
                    n3985 = Boolean To (0,1)(Boolean=w6369) -> (0, 1=w6367:i16)
                    n3986 = Multiply(x=w6367, y=w6368) -> (x*y=w6366:dbl)
                    n3987 = Write to Binary File(file (use dialog)=w6371, data=w6370, 5:w6363, 9:w6365) -> ()  [unwired: 1 in, 4 out]
                    n3988 = Write to Binary File(file (use dialog)=w6364, data=w6366, 5:w6363, 9:w6365) -> ()  [unwired: 2 in, 3 out]
                  }
                }
                n3989 = Greater?(x="Save ave N", y=1.0) -> (0:w6333:bool)
                n3990 = Not(x=w6330) -> (.not. x?=w6332:bool)
                n3991 = And(x=w6332, y=w6333) -> (x .and. y?=w6280:bool)
                n3992 = case shown="True" w6280 {
                  tunnel: w6279 -> [w6344 w6355]
                  tunnel: [w6344 w6347] -> w6278
                  tunnel: "Save ave N" -> [_ w6348]
                  frame False {
                  }
                  frame True {
                    w6345 = 4 ("dimension size")
                    n3993 = Array Size(array=w6355) -> (size(s)=w6349:i32)
                    n3994 = Divide(x=w6349, y=w6345) -> (x/y=w6353:dbl)
                    n3995 = Reshape Array(w6355, w6353, w6345) -> (w6354:u64[][])
                    n3996 = Transpose 2D Array(2D array=w6354) -> (transposed array=w6352:u64[][])
                    n3997 = for {
                      tunnel: w6352 -> [w6357] mode=indexing
                      tunnel: [w6356] -> w6346 mode=indexing
                      tunnel: w6348 -> [w6358]
                      workers-P: _ -> [_]
                      n3998 = call "downsample 1D array - U64.vi"("Ave N"=w6358, "Array In"=w6357) -> ("Array Out"=w6356:u64[])  [unwired: 1 in]
                    }
                    n3999 = Transpose 2D Array(2D array=w6346) -> (transposed array=w6351:u64[][])
                    n4000 = Divide(x=w6349, y=w6348) -> (x/y=w6350:dbl)
                    n4001 = Reshape Array(w6351, w6350) -> (w6347:u64[])
                  }
                }
                n4002 = case shown="True" w6280 {
                  tunnel: w6335 -> [w6372 w6384]
                  tunnel: [w6372 w6376] -> w6331
                  tunnel: "Save ave N" -> [_ w6377]
                  tunnel: w6326 -> [_ w6375]
                  frame False {
                  }
                  frame True {
                    n4003 = Array Size(array=w6384) -> (size(s)=w6378:i32)
                    n4004 = Array Size(array=w6375) -> (size(s)=w6374:i32)
                    n4005 = Divide(x=w6378, y=w6374) -> (x/y=w6382:dbl)
                    n4006 = Reshape Array(w6384, w6382, w6374) -> (w6383:i16[][])
                    n4007 = Transpose 2D Array(2D array=w6383) -> (transposed array=w6381:i16[][])
                    n4008 = for {
                      tunnel: w6381 -> [w6387] mode=indexing
                      tunnel: [w6386] -> w6373 mode=indexing
                      tunnel: w6377 -> [w6385]
                      workers-P: _ -> [_]
                      n4009 = call "downsample 1D array - I16 to F32.vi"("Ave N"=w6385, "Array In"=w6387) -> ("Array Out"=w6386:sgl[])  [unwired: 1 in]
                    }
                    n4010 = Transpose 2D Array(2D array=w6373) -> (transposed array=w6380:sgl[][])
                    n4011 = Divide(x=w6378, y=w6377) -> (x/y=w6379:dbl)
                    n4012 = Reshape Array(w6380, w6379) -> (w6376:sgl[])
                  }
                }
                n4013 = Index Array(array=w6266, index=2) -> (element=w6267:waveform(dbl))
                n4014 = Index Array(array=w6266, index=1) -> (element=w6300:waveform(dbl))
                n4015 = Index Array(array=w6266, index=0) -> (element=w6302:waveform(dbl))
                n4016 = Unbundle By Name(w6267) -> ("Y"=w6269:dbl[])
                n4017 = Unbundle By Name(w6300) -> ("Y"=w6304:dbl[])
                n4018 = Unbundle By Name(w6302) -> ("Y"=w6312:dbl[])
                n4019 = case "Write trap pos. data" shown="True" w6283 {
                  tunnel: w6282 -> [_ w6360]
                  tunnel: w6278 -> [_ w6359]
                  frame False {
                  }
                  frame True {
                    n4020 = Write to Binary File(file (use dialog)=w6360, data=w6359, 5:FALSE ("prepend array or string size? (T)"), 9:T54."big-endian, network order" ("byte order (0:big-endian, network order)")) -> ()  [unwired: 1 in, 4 out]
                  }
                }
                n4021 = Write to Binary File(file (use dialog)=w6338, data=w6331, 5:FALSE ("prepend array or string size? (T)"), 9:T54."big-endian, network order" ("byte order (0:big-endian, network order)")) -> ()  [unwired: 1 in, 4 out]
                n4022 = feedback #33(w6269) -> (w6270:dbl[])
                n4023 = Build Array (concatenate)(w6270, w6269) -> (w6265:dbl[])
                n4024 = Select(t=w6269, s=w6244, f=w6265) -> (s? t:f=w6255:dbl[])
                n4025 = feedback-in #33(w6255) -> ()
                n4026 = feedback #34(w6304) -> (w6306:dbl[])
                n4027 = Build Array (concatenate)(w6306, w6304) -> (w6305:dbl[])
                n4028 = Select(t=w6304, s=w6244, f=w6305) -> (s? t:f=w6294:dbl[])
                n4029 = feedback-in #34(w6294) -> ()
                n4030 = feedback #35(w6312) -> (w6325:dbl[])
                n4031 = Build Array (concatenate)(w6325, w6312) -> (w6324:dbl[])
                n4032 = Select(t=w6312, s=w6244, f=w6324) -> (s? t:f=w6299:dbl[])
                n4033 = feedback-in #35(w6299) -> ()
                n4034 = Divide(x=w6339, y=w6340) -> (x/y=w6342:dbl)
                n4035 = Multiply(x=w6342, y=100.0) -> (x*y=w6341:dbl)
                n4036 = Build Array(w6299, w6294, w6255) -> (→"Saved APD":dbl[][])
                n4037 = Array Size(array=w6299) -> (size(s)=w6317:i32)
                n4038 = Unbundle By Name(w6319) -> ("Y"=w6323:dbl[])
                n4039 = Subtract(x=w6317, y="N pts to average") -> (x-y=w6252:i32)
                n4040 = Multiply(x="N pts to average", y=u16 2) -> (x*y=w6295:u16)
                n4041 = Subtract(x=w6317, y=w6295) -> (x-y=w6253:i32)
                n4042 = feedback #36(w6323) -> (w6322:dbl[])
                n4043 = Build Array (concatenate)(w6322, w6323) -> (w6321:dbl[])
                n4044 = Select(t=w6323, s=w6244, f=w6321) -> (s? t:f=w6320:dbl[])
                "Trap Delta Graph" <- w6320
                n4045 = feedback-in #36(w6320) -> ()
                n4046 = Array Subset(array=w6299, index=w6252, length="N pts to average") -> (w6316:dbl[])
                n4047 = Array Subset(array=w6299, index=w6253, length="N pts to average") -> (w6315:dbl[])
                n4048 = Array Subset(array=w6294, index=w6252, length="N pts to average") -> (w6297:dbl[])
                n4049 = Array Subset(array=w6294, index=w6253, length="N pts to average") -> (w6296:dbl[])
                n4050 = Array Subset(array=w6255, index=w6252, length="N pts to average") -> (w6264:dbl[])
                n4051 = Array Subset(array=w6255, index=w6253, length="N pts to average") -> (w6263:dbl[])
                n4052 = Index Array(array=w6277, index=0) -> (element=w6275:waveform(dbl))
                n4053 = call-poly <vilib>:"Mean.vi"("X"=w6316) -> ("mean"=w6314:dbl)  [unwired: 1 out]
                n4054 = call-poly <vilib>:"Mean.vi"("X"=w6297) -> ("mean"=w6293:dbl)  [unwired: 1 out]
                n4055 = call-poly <vilib>:"Mean.vi"("X"=w6315) -> ("mean"=w6313:dbl)  [unwired: 1 out]
                n4056 = call-poly <vilib>:"Mean.vi"("X"=w6296) -> ("mean"=w6292:dbl)  [unwired: 1 out]
                n4057 = call-poly <vilib>:"Mean.vi"("X"=w6264) -> ("mean"=w6262:dbl)  [unwired: 1 out]
                n4058 = call-poly <vilib>:"Mean.vi"("X"=w6263) -> ("mean"=w6261:dbl)  [unwired: 1 out]
                n4059 = Unbundle By Name(w6275) -> ("Y"=w6273:dbl[])
                n4060 = Subtract(x=w6293, y=w6292) -> (x-y=w6284:dbl)
                "Delta Fl. 2" <- w6284
                n4061 = Subtract(x=w6262, y=w6261) -> (x-y=w6256:dbl)
                "Delta Fl. 3" <- w6256
                n4062 = Subtract(x=w6314, y=w6313) -> (x-y=w6311:dbl)
                "Delta Fl. 1" <- w6311
                n4063 = feedback #37(w6273) -> (w6272:dbl[])
                n4064 = Build Array (concatenate)(w6272, w6273) -> (w6274:dbl[])
                n4065 = Initialize Array(w6311, 1 ("dimension size")) -> (w6308:dbl[])
                n4066 = Initialize Array(w6284, 1 ("dimension size")) -> (w6289:dbl[])
                n4067 = Initialize Array(w6256, 1 ("dimension size")) -> (w6258:dbl[])
                n4068 = Select(t=w6273, s=w6244, f=w6274) -> (s? t:f=w6271:dbl[])
                "Saved trap pos" <- w6271
                n4069 = feedback-in #37(w6271) -> ()
                n4070 = feedback #38(w6308) -> (w6309:dbl[])
                n4071 = Build Array (concatenate)(w6309, w6308) -> (w6307:dbl[])
                n4072 = feedback #39(w6289) -> (w6290:dbl[])
                n4073 = feedback #40(w6258) -> (w6259:dbl[])
                n4074 = Build Array (concatenate)(w6290, w6289) -> (w6288:dbl[])
                n4075 = Build Array (concatenate)(w6259, w6258) -> (w6257:dbl[])
                n4076 = Select(t=w6308, s=w6244, f=w6307) -> (s? t:f=w6287:dbl[])
                n4077 = feedback-in #38(w6287) -> ()
                n4078 = Select(t=w6289, s=w6244, f=w6288) -> (s? t:f=w6286:dbl[])
                n4079 = feedback-in #39(w6286) -> ()
                n4080 = Select(t=w6258, s=w6244, f=w6257) -> (s? t:f=w6251:dbl[])
                n4081 = feedback-in #40(w6251) -> ()
                n4082 = Build Array(w6287, w6286, w6251) -> (→"Save APD Deriv":dbl[][])
                n4083 = Index Array(array=w6243, index=15) -> (element=w6249:waveform(dbl))
                n4084 = Unbundle By Name(w6249) -> ("Y"=w6247:dbl[])
                n4085 = feedback #41(w6247) -> (w6246:dbl[])
                n4086 = Build Array (concatenate)(w6246, w6247) -> (w6248:dbl[])
                n4087 = Select(t=w6247, s=w6244, f=w6248) -> (s? t:f=w6245:dbl[])
                "Amp current" <- w6245
                n4088 = feedback-in #41(w6245) -> ()
              }
            }
            "Progress" <- w6220
            "Progress 2" <- w6220
          }
        }
      }
    }
    n4089 = local read "wait to reset values"() -> (w4946:bool)
    n4090 = Not(x=w4944) -> (.not. x?=w4947:bool)
    n4091 = And(x=w4947, y=w4946) -> (x .and. y?=w4948:bool)
    n4092 = case "Part of MCL raster scanning: returns to initial positions after scan done" shown="True" w4948 {
      tunnel: w4630 -> [w5661 w5668]
      tunnel: [w5661 w5667] -> w4950
      tunnel: w4826 -> [w5660 w5666]
      tunnel: [w5660 w5665] -> w4945
      frame False {
      }
      frame True {
        w5676 = 10.0 ("y")
        w5675 = 32767.0 ("y")
        # "to return scan values\nafter a synchronous \nAOM scan"
        n4093 = local read "AO2"() -> (w5669:dbl)
        n4094 = local read "AO1"() -> (w5670:dbl)
        n4095 = local write "wait to reset values"(FALSE ("wait to reset values")) -> ()
        n4096 = Multiply(x=w5670, y=w5675) -> (x*y=w5672:dbl)
        n4097 = Multiply(x=w5669, y=w5675) -> (x*y=w5674:dbl)
        n4098 = Divide(x=w5672, y=w5676) -> (x/y=w5671:dbl)
        n4099 = Divide(x=w5674, y=w5676) -> (x/y=w5673:dbl)
        n4100 = To Word Integer(number=w5671) -> (16bit integer=w5677:i16)
        n4101 = To Word Integer(number=w5673) -> (16bit integer=w5678:i16)
        n4102 = local read "Total Counts (ticks)"() -> (w5662:u16)
        n4103 = local read "Scan Range (V)\n(of steps)"() -> (w5663:dbl)
        n4104 = xnode "Read/Write Control"("FPGA VI Reference In"=w5668, "error in"=w5666, "AO1 (Y)"=w5677, "AO2 (X)"=w5678, "MCL count"=w5662) -> ("FPGA VI Reference Out"=w5667:T41, "error out"=w5665:errorcluster)
        n4105 = property on="Scan Range (V)\n(of steps)" class="DigNum (strict)"("Val(Sgnl)"=w5663) -> ()  [unwired: 2 in, 2 out]
      }
    }
    n4106 = case shown="True" "Sound ON" {
      tunnel: [w5159 w5204] -> w4792
      tunnel: w4791 -> [w5159 w5203]
      tunnel: w4789 -> [_ _]
      tunnel: w4687 -> [_ w5162]
      tunnel: w4788 -> [_ _]
      tunnel: w4787 -> [_ w5173]
      tunnel: w4786 -> [_ w5183]
      frame False {
      }
      frame True {
        n4107 = Index Array(array=w5162, index="Data channel to sound") -> (element=w5161:waveform(dbl))
        "Waveform Graph 2" <- w5161
        n4108 = Unbundle By Name(w5161) -> ("dt"=w5187:dbl, "Y"=w5185:dbl[])
        n4109 = Array Size(array=w5185) -> (size(s)=w5186:i32)
        "N data samples" <- w5186
        n4110 = for "Data time base" {
          N: w5186 -> [_]
          tunnel: [w5208] -> w5188 mode=indexing
          i -> [w5208]
        }
        n4111 = Multiply(x=w5187, y=w5188) -> (x*y=w5184:dbl[])
        n4112 = Compound Arithmetic op=MULTIPLY(6.283185307179586, "Carrier Frequency (Hz)", w5183) -> (w5200:dbl[])
        n4113 = call <vilib>:"Interpolate 1D.vi"("X is monotonic"=TRUE, "xi"=w5183, "X"=w5184, "Y"=w5185) -> ("yi"=w5181:dbl[])  [unwired: 5 in, 2 out]
        n4114 = Sine(x=w5200) -> (sin(x)=w5189:dbl[])
        n4115 = Add(x=w5181, y="Offset") -> (x+y=w5179:dbl[])
        n4116 = Multiply(x=w5179, y="mult x") -> (x*y=w5177:dbl[])
        n4117 = Add(x="Offset 2", y=w5177) -> (x+y=w5172:dbl[])
        n4118 = Compound Arithmetic op=MULTIPLY(6.283185307179586, "Carrier Frequency (Hz)", w5173, w5172) -> (w5164:dbl[])
        n4119 = for "Cumulative sum" {
          tunnel: [w5207] -> w5170 mode=indexing
          shift-right: [w5207] -> w5167
          shift-left: 0.0 -> [w5206]
          tunnel: w5164 -> [w5205] mode=indexing
          n4120 = Add(x=w5205, y=w5206) -> (x+y=w5207:dbl)
        }
        n4121 = feedback #42(0.0) -> (w5166:dbl)
        n4122 = Add(x=w5170, y=w5166) -> (x+y=w5169:dbl[])
        n4123 = Add(x=w5167, y=w5166) -> (x+y=w5165:dbl)
        n4124 = feedback-in #42(w5165) -> ()
        n4125 = Sine(x=w5169) -> (sin(x)=w5163:dbl[])
        n4126 = Select(t=w5189, s="tone or data", f=w5163) -> (s? t:f=w5195:dbl[])
        n4127 = Multiply(x=w5195, y="Volume") -> (x*y=w5193:dbl[])
        n4128 = Initialize Array(0.0 ("element"), "N initial buffer elements") -> (w5196:dbl[])
        n4129 = Multiply(x="N initial buffer elements", y=w5173) -> (x*y=→"Initial buffer time (s)":dbl)
        n4130 = Build Array (concatenate)(w5196, w5193) -> (w5198:dbl[])
        n4131 = First Call?() -> (First Call?: T/F=w5199:bool)
        n4132 = Select(t=w5198, s=w5199, f=w5193) -> (s? t:f=w5192:dbl[])
        n4133 = call-poly <vilib>:"Sound Output Write.vi"("data"=w5192, "task ID"=w5203) -> ("task ID out"=w5204:T61)  [unwired: 8 in, 1 out]
      }
    }
    n4134 = node-c288() -> ()  [unwired: 2 out]
  }
  n4135 = disable-structure shown="Disabled" {
    disable-tunnel: w21 -> [w6388 _]
    frame Disabled {
      n4136 = call <vilib>:"Sound Output Clear.vi"("task ID"=w6388) -> ()  [unwired: 10 in, 1 out]
    }
    frame Enabled {
    }
  }
  n4137 = node-c288(w59) -> ()  [unwired: 1 out]
  n4138 = node-c288(w67) -> ()  [unwired: 1 out]
  n4139 = flat-sequence {
    tunnel: w74 -> [w6392]
    tunnel: w75 -> [w6393]
    tunnel: [w6391] -> w73
    tunnel: [w6390] -> w72
    tunnel: w71 -> [_]
    tunnel: w69 -> [_]
    tunnel: w65 -> [_]
    tunnel: w73 -> [w6394]
    tunnel: w72 -> [w6395]
    frame #0 {
      w6389 = FALSE ("AI to FIFO")
      n4140 = xnode "Read/Write Control"("FPGA VI Reference In"=w6393, "error in"=w6392, "AI to FIFO"=w6389, "APD to FIFO"=w6389) -> ("FPGA VI Reference Out"=w6391:T41, "error out"=w6390:errorcluster)
    }
    frame #1 {
      n4141 = xnode "Close FPGA VI Reference"("FPGA VI Reference In"=w6394, "error in"=w6395) -> ("error out"=→"error out":errorcluster)
    }
  }
